vi "UHR-Fleezers Control (host) - Avogadro v3.vi"() -> ()   [LabVIEW 2014] (continued)
            n3132 = call "Calculate MCL scan parameters.vi"("Input parameters"=w5700) -> ("Scan steps(MCL)"=w5699:dbl, "Scan Freq. Increment (MCL)"=w5698:dbl, "MCL Count"=w5697:dbl)
            "MCL Count" <- w5697
            n3133 = xnode "Read/Write Control"("FPGA VI Reference In"=w5714, "error in"=w5713, "Scan steps (MCL)"=w5699, "Number of scans (MCL)"=w5710, "Cycles per step (MCL)"=u64 1, "Scan freq.  increment (MCL)"=w5698, "1D or 2D Scan?"=w5711, "MCL Scan Axis"=w5711, "Cont. Scan (MCL)"=w5711, "MCL count"=w5697) -> ("FPGA VI Reference Out"=w5696:T41, "error out"=w5712:errorcluster)
            n3134 = local write "MCL Scanning"(w5715) -> ()
            n3135 = local write "wait to reset values"(w5715) -> ()
            n3136 = xnode "Read/Write Control"("FPGA VI Reference In"=w5696, "error in"=w5712, "AI to FIFO"=w5715, "APD to FIFO"=w5715, "Start scan"=w5715, "Start scan (MCL)"=w5715) -> ("FPGA VI Reference Out"=w5717:T41, "error out"=w5716:errorcluster)
          }
        }
        "Raster Scanning..." <- TRUE ("Scanning...")
      }
    }
    n3137 = case "Start MCL raster scan" shown="True" w4761 {
      tunnel: w4926 -> [w5558 w5576]
      tunnel: w4925 -> [w5557 w5575]
      tunnel: [w5558 w5571] -> w4877
      tunnel: [w5557 w5570] -> w4876
      tunnel: [FALSE w5569] -> w4909
      tunnel: "Start MCL Scan" -> [_ w5566]
      tunnel: "Confocal Image" -> [_ w5565]
      tunnel: "Confocal Linescan" -> [_ _]
      frame False {
      }
      frame True {
        w5569 = TRUE
        n3138 = case shown="True" "Restart DMA? (MCL)" {
          tunnel: [w5652 w5654] -> w5574
          tunnel: [w5651 w5653] -> w5573
          tunnel: w5576 -> [w5652 w5657]
          tunnel: w5575 -> [w5651 w5656]
          frame False {
          }
          frame True {
            n3139 = call "reset FPGA DMA.vi"("error in"=w5656, "FPGA VI Reference In"=w5657) -> ("error out"=w5653:errorcluster, "FPGA VI Reference Out"=w5654:T41)
            n3140 = local write "Overflow (data lost)"(FALSE ("Overflow (data lost)")) -> ()
          }
        }
        n3141 = case shown="False" w5566 {
          tunnel: w5565 -> [w5579 _]
          frame False {
            n3142 = property on="Confocal Image" class="Bool (strict)"("Value"=FALSE ("Start Confocal Map")) -> ()  [unwired: 2 in, 2 out]
            n3143 = property on="2D or 1D Scan" class="Bool (strict)"("Val(Sgnl)"=w5579) -> ()  [unwired: 2 in, 2 out]
          }
          frame True {
          }
        }
        n3144 = local write "Tab Control 6"(T63."Imaging" ("Tab Control 6")) -> ()
        n3145 = local read "T3 X (V)"() -> (w5561:dbl)
        n3146 = local write "MCL Scanning"(w5569) -> ()
        n3147 = local read "T3 Y (V)"() -> (w5560:dbl)
        n3148 = local read "AO2"() -> (w5562:dbl)
        n3149 = local read "AO1"() -> (w5563:dbl)
        n3150 = case shown="True" "Center Scan" {
          tunnel: w5574 -> [w5592 w5614]
          tunnel: w5573 -> [w5591 w5613]
          tunnel: [w5590 w5612] -> w5571
          tunnel: [w5589 w5611] -> w5570
          tunnel: [w5584 w5608] -> w5568
          tunnel: [w5585 w5607] -> w5567
          tunnel: w5563 -> [w5582 w5610]
          tunnel: w5562 -> [w5581 w5609]
          tunnel: "Scan trap 3 or Fl?" -> [w5587 w5606]
          tunnel: w5561 -> [w5586 w5599]
          tunnel: w5560 -> [w5583 w5600]
          frame False {
            w5588 = TRUE ("AI to FIFO")
            n3151 = case shown="False" w5587 {
              tunnel: [w5594 w5598] -> w5585
              tunnel: w5586 -> [_ w5598]
              tunnel: [w5595 w5597] -> w5584
              tunnel: w5583 -> [_ w5597]
              tunnel: w5582 -> [w5595 _]
              tunnel: w5581 -> [w5594 _]
              tunnel: [FALSE ("AI to FIFO") TRUE ("AI to FIFO")] -> w5580
              frame False {
              }
              frame True {
              }
            }
            n3152 = xnode "Read/Write Control"("FPGA VI Reference In"=w5592, "error in"=w5591, "AI to FIFO"=w5588, "APD to FIFO"=w5588, "Start scan (MCL)"=w5588, "ScanTrap 3 or Fl-laser"=w5580) -> ("FPGA VI Reference Out"=w5590:T41, "error out"=w5589:errorcluster)
          }
          frame True {
            n3153 = local read "Actual MCL Inc (V)"() -> (w5601:dbl)
            n3154 = local read "Scan steps (MCL)"() -> (w5602:u64)
            n3155 = local read "Scan lines (y)"() -> (w5603:u64)
            n3156 = local read "Fast Scan Dir"() -> (w5604:bool)
            n3157 = local read "2D or 1D Scan"() -> (w5605:bool)
            n3158 = case shown="False" w5606 {
              tunnel: w5614 -> [w5632 w5650]
              tunnel: w5613 -> [w5631 w5649]
              tunnel: [w5630 w5648] -> w5612
              tunnel: [w5629 w5647] -> w5611
              tunnel: w5610 -> [w5625 _]
              tunnel: w5609 -> [w5624 _]
              tunnel: [w5622 w5642] -> w5608
              tunnel: [w5621 w5641] -> w5607
              tunnel: w5605 -> [w5620 w5640]
              tunnel: w5604 -> [w5619 w5639]
              tunnel: w5603 -> [w5618 w5638]
              tunnel: w5602 -> [w5617 w5637]
              tunnel: w5601 -> [w5615 w5635]
              tunnel: w5600 -> [_ w5634]
              tunnel: w5599 -> [_ w5633]
              frame False {
                w5628 = TRUE ("AI to FIFO")
                n3159 = Bundle("Actual MCL Inc (V)"=w5615, "Scan steps (MCL)"=w5617, "Scan lines (y)"=w5618, "AO1"=w5625, "AO2"=w5624) -> (w5623:T67)  [unwired: 1 in]
                n3160 = call "Center Scan calculation.vi"("2D or 1D Scan"=w5620, "Fast Scan Dir"=w5619, "Input parameters"=w5623) -> ("X"=w5621:dbl, "Y"=w5622:dbl)
                n3161 = call "Volt to I16.vi"("Voltage In"=w5622) -> ("I16 Voltage Out"=w5627:i16)
                n3162 = call "Volt to I16.vi"("Voltage In"=w5621) -> ("I16 Voltage Out"=w5626:i16)
                n3163 = xnode "Read/Write Control"("FPGA VI Reference In"=w5632, "error in"=w5631, "AI to FIFO"=w5628, "APD to FIFO"=w5628, "Start scan (MCL)"=w5628, "AO1 (Y)"=w5627, "AO2 (X)"=w5626, "ScanTrap 3 or Fl-laser"=FALSE ("AI to FIFO")) -> ("FPGA VI Reference Out"=w5630:T41, "error out"=w5629:errorcluster)
              }
              frame True {
                w5646 = TRUE ("AI to FIFO")
                n3164 = Bundle("Actual MCL Inc (V)"=w5635, "Scan steps (MCL)"=w5637, "Scan lines (y)"=w5638, "T3 Y (V)"=w5634, "T3 X (V)"=w5633) -> (w5643:T68)  [unwired: 1 in]
                n3165 = call "Center Scan calculation.vi"("2D or 1D Scan"=w5640, "Fast Scan Dir"=w5639, "Input parameters"=w5643) -> ("X"=w5641:dbl, "Y"=w5642:dbl)
                n3166 = call "Volt to I16.vi"("Voltage In"=w5642) -> ("I16 Voltage Out"=w5645:i16)
                n3167 = call "Volt to I16.vi"("Voltage In"=w5641) -> ("I16 Voltage Out"=w5644:i16)
                n3168 = xnode "Read/Write Control"("FPGA VI Reference In"=w5650, "error in"=w5649, "AI to FIFO"=w5646, "APD to FIFO"=w5646, "Start scan (MCL)"=w5646, "Piezo Trap Y (AO4)"=w5645, "Piezo Trap X (AO5)"=w5644, "ScanTrap 3 or Fl-laser"=TRUE ("AI to FIFO")) -> ("FPGA VI Reference Out"=w5648:T41, "error out"=w5647:errorcluster)
              }
            }
          }
        }
        "Initial Y" <- w5568
        "Initial X" <- w5567
        "wait to reset values" <- w5569
      }
    }
    n3169 = xnode "Read/Write Control"("FPGA VI Reference In"=w4738) -> ("FPGA VI Reference Out"=w4633:T41, "BD1 Frequency Out 1"=w4740:u64, "Piezo X out"=w4672:i16, "Piezo Y out"=w4671:i16)  [unwired: 1 in, 1 out]
    n3170 = And(x="Save scans", y=w4906) -> (x .and. y?=w4924:bool)
    n3171 = call "IR AOM word to freq.vi"("Frequency Word In (U64)"=w4740) -> ("Frequency Out (MHz)"=w4739:dbl)
    n3172 = Divide(x=w4672, y=w4706) -> (x/y=w4705:dbl)
    n3173 = Divide(x=w4671, y=w4706) -> (x/y=w4704:dbl)
    n3174 = local read "BD 1 Frequency 2 (MHz)"() -> (w4770:dbl)
    n3175 = Subtract(x=w4770, y=w4739) -> (x-y=w4703:dbl)
    "Current deltaF (MHz)" <- w4703
    n3176 = Build Array(w4703, w4705, w4704) -> (w4629:dbl[])
    "Trap position array" <- w4629
    n3177 = control-ref of="Piezo trap cursor control"() -> (w4712:refnum<vi>)
    n3178 = Unbundle By Name("Cursor control") -> ("X"=w4714:bool, "Y"=w4713:bool)
    n3179 = local read "APD Elements/DMA read"() -> (w4801:u32)
    n3180 = local read "Trap AI Elements/DMA read"() -> (w4898:u32)
    n3181 = case shown="False" w4714 {
      tunnel: w4712 -> [w5061 w5071]
      tunnel: w4633 -> [_ w5063]
      frame False {
        n3182 = local read "T3 X (V)"() -> (w5062:dbl)
        n3183 = property class="XYGraph (strict)"(reference=w5061, "Cursor.Cursor X"=w5062) -> ()  [unwired: 1 in, 2 out]
      }
      frame True {
        n3184 = property class="XYGraph (strict)"(reference=w5071) -> ("Cursor.Cursor X"=w5068:dbl)  [unwired: 1 in, 2 out]
        n3185 = In Range and Coerce(upper limit=10.0, x=w5068, lower limit=0.0) -> (coerced(x)=w5066:dbl)  [unwired: 1 out]
        n3186 = Multiply(x=3276.7, y=w5066) -> (x*y=w5065:dbl)
        n3187 = To Unsigned Word Integer(number=w5065) -> (unsigned 16bit integer=w5064:u16)
        n3188 = xnode "Read/Write Control"("FPGA VI Reference In"=w5063, "Piezo Trap X (AO5)"=w5064) -> ()  [unwired: 1 in, 2 out]
      }
    }
    n3189 = case shown="False" w4713 {
      tunnel: w4712 -> [w5048 w5060]
      tunnel: w4633 -> [_ w5051]
      frame False {
        n3190 = local read "T3 Y (V)"() -> (w5050:dbl)
        n3191 = Negate(x=w5050) -> (-x=w5049:dbl)
        n3192 = property class="XYGraph (strict)"(reference=w5048, "Cursor.Cursor Y"=w5049) -> ()  [unwired: 1 in, 2 out]
      }
      frame True {
        n3193 = property class="XYGraph (strict)"(reference=w5060) -> ("Cursor.Cursor Y"=w5057:dbl)  [unwired: 1 in, 2 out]
        n3194 = In Range and Coerce(upper limit=0.0, x=w5057, lower limit=-10.0) -> (coerced(x)=w5056:dbl)  [unwired: 1 out]
        n3195 = Negate(x=w5056) -> (-x=w5054:dbl)
        n3196 = Multiply(x=3276.7, y=w5054) -> (x*y=w5053:dbl)
        n3197 = To Unsigned Word Integer(number=w5053) -> (unsigned 16bit integer=w5052:u16)
        n3198 = xnode "Read/Write Control"("FPGA VI Reference In"=w5051, "Piezo Trap Y (AO4)"=w5052) -> ()  [unwired: 1 in, 2 out]
      }
    }
    n3199 = local read "Trap Pos Elements/DMA read"() -> (w4873:u32)
    n3200 = local read "DMA Update Period (s)"() -> (w4754:dbl)
    n3201 = xnode "Invoke Method"("FPGA VI Reference In"=w4877, "error in"=w4876, "Number of Elements"=w4873, "Timeout (ms)"=-1) -> ("Data"=w4709:u16[], "Elements Remaining"=→"Trap Pos FIFO El Remaining":u32)  [unwired: 2 out]
    n3202 = xnode "Get Trap Data"("FPGA VI Reference In"=w4877, "error in"=w4876, "Number of Elements"=w4898, "Timeout (ms)"=-1 ("Timeout")) -> ("FPGA VI Reference Out"=w4769:T41, "error out"=w4825:errorcluster, "Data"=w4758:i16[], "Elements Remaining"=w4958:u32)
    "FIFO El. Rem." <- w4958
    n3203 = local read "Trap AI FIFO Depth"() -> (w4960:u32)
    n3204 = xnode "Get APD Data"("FPGA VI Reference In"=w4877, "error in"=w4876, "Number of Elements"=w4801, "Timeout (ms)"=-1) -> ("Data"=w4750:u32[], "Elements Remaining"=→"APD FIFO Elements Remaining":u32)  [unwired: 2 out]
    n3205 = feedback #1(0.0) -> (w4871:dbl)
    n3206 = To Time Stamp(1:w4871) -> (0:w4653:timestamp)
    n3207 = Add(x=w4754, y=w4871) -> (x+y=w4935:dbl)
    n3208 = feedback-in #1(w4935) -> ()
    n3209 = Subtract(x=w4960, y=w4898) -> (x-y=w4959:u32)
    n3210 = local read "APD Integration Time (s)"() -> (w4742:dbl)
    n3211 = local read "Scan trap 3 or Fl?"() -> (w4628:bool)
    n3212 = Divide(x=w4958, y=w4959) -> (x/y=w4957:dbl)
    "Buffer Status" <- w4957
    n3213 = local read "Trap Sets"() -> (w4759:u32)
    n3214 = Equal?(x=w4957, y=1.0) -> (x = y?=w4955:bool)
    n3215 = local read "Number of APDs"() -> (w4749:u8)
    n3216 = case "Alert buffer overflow" shown="True" w4955 {
      frame False {
      }
      frame True {
        n3217 = call <vilib>:"Beep.vi"() -> ()  [unwired: 3 in, 9 out]
        "Overflow (data lost)" <- TRUE ("Overflow (data lost)")
      }
    }
    n3218 = call "deinterlace.vi"("Scan trap 3 or Fl?"=w4628, "Detector type"="Detector Type", "Data"=w4758, "Trap sets"=w4759, "Flip x sign"="Flip X Sign") -> ("Channel pattern"=w4755:i32, "Channel names"=w4711:string[], "Deinterlaced normalized data"=w4647:dbl[][], "Deinterlaced data"=w4756:i16[])
    "AI labels" <- w4711
    n3219 = local read "Data Period (s)"() -> (w4646:dbl)
    n3220 = call "Trap_position_vectors.vi"("Data array"=w4709) -> ("Output data for plotting"=w4708:dbl[][], "Output data for saving"=w4707:u64[])
    n3221 = call "APD data extraction.vi"("Data"=w4750, "Number of APD's"=w4749, "APD integration time (s)"=w4742, "APD Ave N"="APD Ave N", "APD Disp. Downsample"="APD Disp. Downsample", "APD Disp. Scale"="APD Disp. Scale", "Time Stamp"=w4653) -> ("Output cluster"=→"APD rates cluster":T2, "Output Data"=w4745:T69, "Output waveform"=w4744:waveform(dbl)[], "APD Display period (s)"=w4743:dbl)
    "APD Display Period (s)" <- w4743
    n3222 = Reciprocal(x=w4743) -> (1/x=→"APD Display Freq. (Hz)":dbl)
    n3223 = Multiply(x=w4646, y="Trap Disp. Downsample") -> (x*y=w4872:dbl)
    "Display Period (s)" <- w4872
    n3224 = for {
      tunnel: w4647 -> [w5086] mode=indexing
      tunnel: [w5085] -> w4710 mode=indexing
      n3225 = call-poly <vilib>:"Mean.vi"("X"=w5086) -> ("mean"=w5085:dbl)  [unwired: 1 out]
    }
    "Values" <- w4710
    n3226 = Decimate 1D Array(w4756) -> (w4863:i16[], w4862:i16[], w4860:i16[], w4859:i16[])  [unwired: 9 out]
    n3227 = call "Generate Waveform.vi"("Downsampling"="Trap Disp. Downsample", "Data Period (s)"=w4646, "Data"=w4647, "Plot names"=w4711, "Time Stamp"=w4653) -> ("Downsampled data"=w4689:waveform(dbl)[], "Non downsampled waveform"=w4751:waveform(dbl)[])
    n3228 = Multiply(x="APD Disp. Scale", y=w4744) -> (x*y=w4881:waveform(dbl)[])
    n3229 = Reciprocal(x=w4872) -> (1/x=→"Trap Disp. Freq. (Hz)":dbl)
    n3230 = Multiply(x="APD Disp. Downsample", y=w4742) -> (x*y=w4880:dbl)
    n3231 = Divide(x=w4863, y=w4862) -> (x/y=w4864:dbl[])
    n3232 = Divide(x=w4860, y=w4859) -> (x/y=w4861:dbl[])
    n3233 = Divide(x=w4881, y=w4880) -> (x/y=w4805:waveform(dbl)[])
    n3234 = case shown="1" "Plot Trap Positions" {
      tunnel: [w5072 w5080] -> w4733
      frame 0, Default {
        n3235 = local read "BD 1 Frequency 2 (MHz)"() -> (w5075:dbl)
        n3236 = local read "BD 1 Frequency 1 (MHz)"() -> (w5076:dbl)
        n3237 = local read "T3 Y (V)"() -> (w5073:dbl)
        n3238 = local read "T3 X (V)"() -> (w5074:dbl)
        n3239 = Build Array(w5076, w5075, w5074, w5073) -> (w5072:dbl[])
      }
      frame 1 {
        w5079 = 60.0
        n3240 = local read "Piezo trap x\noffset (V)"() -> (w5077:dbl)
        n3241 = Build Array(w5079, w5079, w5077, "Piezo trap y\noffset (V)") -> (w5080:dbl[])
      }
    }
    n3242 = Split 1D Array(array=w4864, index="N El. to Ave.") -> (second subarray=w4867:dbl[])  [unwired: 1 out]
    n3243 = Split 1D Array(array=w4861, index="N El. to Ave.") -> (second subarray=w4866:dbl[])  [unwired: 1 out]
    n3244 = case shown="True" "Chart APD?" {
      tunnel: w4805 -> [_ w5026]
      frame False {
      }
      frame True {
        n3245 = Index Array(array=w5026, index=0) -> (element=w5036:waveform(dbl))
        n3246 = Index Array(array=w5026, index=1) -> (element=w5034:waveform(dbl))
        n3247 = Index Array(array=w5026, index=2) -> (element=w5028:waveform(dbl))
        n3248 = Subtract(x=w5036, y="APD 1 Offset") -> (x-y=w5032:waveform(dbl))
        n3249 = Subtract(x=w5034, y="APD 2 Offset") -> (x-y=w5031:waveform(dbl))
        n3250 = Subtract(x=w5028, y="APD 3 Offset") -> (x-y=w5025:waveform(dbl))
        n3251 = Build Array(w5032, w5031, w5025) -> (→"APD Chart":waveform(dbl)[])
      }
    }
    n3252 = local read "AOM X Cal (nm/MHz)"() -> (w4735:dbl)
    n3253 = call-poly <vilib>:"Mean.vi"("X"=w4867) -> ("mean"=w4855:dbl)  [unwired: 1 out]
    n3254 = call-poly <vilib>:"Mean.vi"("X"=w4866) -> ("mean"=w4854:dbl)  [unwired: 1 out]
    n3255 = local read "Trap X AI1 (DMA)"() -> (w4865:T23)
    n3256 = To Fixed-Point(number=w4854) -> (fixed-point=w4852:fxp<+/-,16,1>)  [unwired: 1 in]
    n3257 = To Fixed-Point(number=w4855) -> (fixed-point=w4853:fxp<+/-,16,1>)  [unwired: 1 in]
    n3258 = Bundle By Name(cluster=w4865, "Set 1"=w4853, "Set 2"=w4852) -> (→"Trap X AI1 (DMA)":T23)
    n3259 = Build Array(w4735, w4735, "Piezo Trap X cal (nm/V)", "Piezo Trap Y cal (nm/V)") -> (w4734:dbl[])
    n3260 = Cluster To Array(cluster="Negate Axis") -> (array=w4728:bool[])
    n3261 = call "Generate Trap Positiion Waveform.vi"("Base trap positions"=w4733, "Data Period (s)"=w4646, "Input data"=w4708, "Position calibration values"=w4734, "Trap Pos. Disp. Downsample (s)"="Trap Pos. Disp. Downsample", "Negate axis"=w4728, "Time Stamp"=w4653) -> ("Output waveforms"=w4716:waveform(dbl)[], "Output trap positions"=w4662:cluster{"X":dbl[], "Y":dbl[]}[])  [unwired: 2 in]
    "Trap Positions" <- w4716
    n3262 = Initialize Array(0.0) -> (w4730:dbl[][])  [unwired: 2 in]
    n3263 = local read "Display Period (s)"() -> (w4889:dbl)
    n3264 = for {
      tunnel: w4716 -> [w5084] mode=indexing
      shift-right: [w5082] -> w4718
      shift-left: w4730 -> [w5083]
      n3265 = Unbundle By Name(w5084) -> ("Y"=w5081:dbl[])
      n3266 = Build Array (concatenate)(w5083, w5081) -> (w5082:dbl[][])
    }
    n3267 = Build Array (concatenate)(w4744, w4689) -> (w4753:waveform(dbl)[])
    "All Signals" <- w4753
    n3268 = Initialize Array(0.0) -> (w4643:dbl[][])  [unwired: 2 in]
    n3269 = feedback #2(w4643) -> (w4642:dbl[][])
    n3270 = Divide(x="Bead Sep. Int. Time (s)", y=w4889) -> (x/y=w4724:dbl)
    n3271 = case shown="True" "Start position \nscan" {
      tunnel: w4642 -> [w5039 _]
      tunnel: [w5039 w5047] -> w4641
      tunnel: "T3 positioning test range (V)" -> [_ w5041]
      frame False {
      }
      frame True {
        n3272 = local read "BD 1 Frequency 1 (MHz)"() -> (→"AOM position for scan (MHz)":dbl)
        n3273 = Unbundle By Name(w5041) -> ("Xmin"=w5043:dbl, "Ymin"=w5042:dbl)
        n3274 = local write "Start position \nscan"(FALSE) -> ()
        n3275 = local write "T3 X (V)"(w5043) -> ()
        n3276 = local write "T3 Y (V)"(w5042) -> ()
        n3277 = Initialize Array(0.0) -> (w5047:dbl[][])  [unwired: 2 in]
        "Position\nscanning..." <- TRUE
      }
    }
    n3278 = case shown="True" "Measure \ncorrelation?" {
      tunnel: w4647 -> [_ w5013]
      tunnel: w4646 -> [_ w5012]
      tunnel: w4641 -> [w4983 w4996]
      tunnel: [w4983 w4989] -> w4640
      tunnel: "T3 positioning test range (V)" -> [_ w4988]
      tunnel: w4633 -> [_ w4984]
      frame False {
      }
      frame True {
        n3279 = local read "DMA Update Period (s)"() -> (w4991:dbl)
        n3280 = Divide(x="Correlation integration time (s)", y=w4991) -> (x/y=w4990:dbl)
        n3281 = To Word Integer(number=w4990) -> (16bit integer=w4986:i16)
        n3282 = Divide(x="Correlation integration time (s)", y=w5012) -> (x/y=w5006:dbl)
        n3283 = Initialize Array(0.0, w5006, 4) -> (w5009:dbl[][])
        n3284 = feedback #3(w5009) -> (w5008:dbl[][])
        n3285 = call "correlation calculation for trap 3 absolute positioning.vi"("Number of sets to average"=w5006, "Accumulated array"=w5008, "raw data"=w5013) -> ("Accumulated array out"=w5007:dbl[][], "Y correlation"=w5004:dbl, "X correlation"=w5005:dbl)
        "3-1 x correlation" <- w5005
        "3-1 y correlation" <- w5004
        n3286 = feedback-in #3(w5007) -> ()
        n3287 = Increment(x=w4986) -> (x+1=w4985:i16)
        n3288 = local read "Position\nscanning..."() -> (w4995:bool)
        n3289 = Bundle("X correlation"=w5005, "Y correlation"=w5004) -> (w5003:T70)  [unwired: 1 in]
        n3290 = local read "T3 Y (V)"() -> (w5001:dbl)
        n3291 = local read "T3 X (V)"() -> (w5002:dbl)
        n3292 = Bundle("T3 X (V)"=w5002, "T3 Y (V)"=w5001) -> (w5000:cluster{"T3 X (V)":dbl, "T3 Y (V)":dbl})  [unwired: 1 in]
        n3293 = feedback #4(i16 0) -> (w4998:i16)
        n3294 = call "correlation scan.vi"("Correlations in"=w5003, "Voltages in"=w5000, "Cycle counter"=w4998, "in put Array"=w4996, "T3 positioning \ntest range (V)"=w4988, "Number of acquisition cycles"=w4985, "Scanning?"=w4995) -> ("Voltages out"=w4993:cluster{"X":dbl, "Y":dbl}, "Scanning out"=w4994:bool, "Output array"=w4989:dbl[][], "Cycle counter out"=w4997:i16)
        n3295 = feedback-in #4(w4997) -> ()
        n3296 = local write "Position\nscanning..."(w4994) -> ()
        n3297 = case shown="True" w4994 {
          tunnel: w4993 -> [_ w5024]
          tunnel: w4984 -> [_ w5018]
          frame False {
          }
          frame True {
            w5022 = 3276.7
            n3298 = Unbundle By Name(w5024) -> ("X"=w5023:dbl, "Y"=w5021:dbl)
            n3299 = Multiply(x=w5022, y=w5023) -> (x*y=w5020:dbl)
            n3300 = Multiply(x=w5022, y=w5021) -> (x*y=w5019:dbl)
            n3301 = To Word Integer(number=w5020) -> (16bit integer=w5017:i16)
            n3302 = To Word Integer(number=w5019) -> (16bit integer=w5016:i16)
            n3303 = local write "T3 Y (V)"(w5021) -> ()
            n3304 = local write "T3 X (V)"(w5023) -> ()
            n3305 = xnode "Read/Write Control"("FPGA VI Reference In"=w5018, "Piezo Trap X (AO5)"=w5017, "Piezo Trap Y (AO4)"=w5016) -> ()  [unwired: 1 in, 2 out]
          }
        }
        n3306 = case shown="True" "Stop scan" {
          frame False {
          }
          frame True {
            n3307 = local write "Position\nscanning..."(FALSE) -> ()
            n3308 = local write "Stop scan"(FALSE) -> ()
          }
        }
      }
    }
    n3309 = feedback-in #2(w4640) -> ()
    n3310 = feedback #5(w4718) -> (w4725:dbl[][])
    n3311 = call "Trap Pos RMS.vi"("Accumulated array"=w4725, "New Array"=w4718, "Number of sets to average"=w4724) -> ("Output accumulated array"=w4723:dbl[][], "RMS"=w4721:dbl[], "Mean"=w4722:dbl[])
    n3312 = feedback-in #5(w4723) -> ()
    n3313 = Index Array(array=w4718, index (row)=0 ("index")) -> (element=w4717:dbl[])  [unwired: 1 in]
    n3314 = local read "Two Trap Offset Values"() -> (w4699:T32)
    n3315 = Array To Cluster(array=w4721) -> (cluster=→"Trap RMS (ang)":T71)
    n3316 = Array To Cluster(array=w4722) -> (cluster=→"Mean Trap Positions (nm)":T72)
    n3317 = local read "MCL offset scanning range (V)"() -> (w4697:T4)
    n3318 = local read "Multi-MCL offset array"() -> (w4698:T31)
    n3319 = local read "Multiple-MCL offset?"() -> (w4702:bool)
    n3320 = local read "Offset file step size"() -> (w4700:dbl)
    n3321 = local read "T1 calibration"() -> (w4696:T12)
    n3322 = local read "T2 calibration"() -> (w4695:T12)
    n3323 = local read "T3 calibration"() -> (w4694:T12)
    n3324 = local read "Trap Disp. Downsample"() -> (w4651:dbl)
    n3325 = Build Array(w4696, w4695, w4694) -> (w4693:T56)
    n3326 = call "calibrate trap data V3RG.vi"("array of calibration clusters"=w4693, "Trap position array"=w4629, "MCL offset scanning range (V)"=w4697, "Multi-MCL offset array"=w4698, "two trap offset values"=w4699, "Dynamic offset update"="Dynamic offset\nupdate", "Multiple-MCL offset?"=w4702, "x (true) or y (false)"=TRUE, "Data array"=w4689, "Offset File step size"=w4700) -> ("Positions out"=w4691:dbl[][], "Forces out (pN)"=w4690:dbl[][])
    n3327 = local read "Mean Trap Positions (nm)"() -> (w4688:T6)
    n3328 = local read "Trap 2 Bead Size (nm)"() -> (w4666:dbl)
    n3329 = local read "Trap 3 Bead Size (nm)"() -> (w4665:dbl)
    n3330 = local read "Trap 1 Bead Size (nm)"() -> (w4667:dbl)
    n3331 = case shown="True" "Measure \ncorrelation?" {
      tunnel: w4640 -> [_ w4967]
      tunnel: "T3 positioning test range (V)" -> [_ w4966]
      frame False {
      }
      frame True {
        n3332 = Unbundle By Name(w4966) -> ("Xmax"=w4970:dbl, "Xmin"=w4971:dbl, "increment"=w4976:dbl, "Ymax"=w4972:dbl, "Ymin"=w4973:dbl)
        n3333 = Index Array(array=w4967, index (col)=3) -> (element=w4969:dbl[])  [unwired: 1 in]
        n3334 = Index Array(array=w4967, index (col)=2) -> (element=w4968:dbl[])  [unwired: 1 in]
        n3335 = Subtract(x=w4972, y=w4973) -> (x-y=w4975:dbl)
        n3336 = Subtract(x=w4970, y=w4971) -> (x-y=w4974:dbl)
        n3337 = Quotient & Remainder(x=w4975, y=w4976) -> (floor(x/y)=w4978:dbl)  [unwired: 1 out]
        n3338 = Quotient & Remainder(x=w4974, y=w4976) -> (floor(x/y)=w4977:dbl)  [unwired: 1 out]
        n3339 = Increment(x=w4977) -> (x+1=w4980:dbl)
        n3340 = Increment(x=w4978) -> (x+1=w4979:dbl)
        n3341 = Reshape Array(w4969, w4980, w4979) -> (→"Correlations in Y":dbl[][])
        n3342 = Reshape Array(w4968, w4980, w4979) -> (→"Correlations in X":dbl[][])
      }
    }
    n3343 = local read "Data Period (s)"() -> (w4655:dbl)
    n3344 = Index Array(array=w4689, index="index 2") -> (element=w4800:waveform(dbl))
    n3345 = Index Array(array=w4689, index="index 1") -> (element=w4796:waveform(dbl))
    n3346 = Multiply(x=w4651, y=w4655) -> (x*y=w4654:dbl)
    n3347 = Unbundle By Name(w4800) -> ("Y"=w4799:dbl[])
    n3348 = Unbundle By Name(w4796) -> ("Y"=w4795:dbl[])
    n3349 = Build Array(w4667, w4666, w4665) -> (w4664:dbl[])
    n3350 = call "Force and position waveforms.vi"("Input waveforms"=w4689, "Forces  (pN)"=w4690, "Deflections (nm)"=w4691, "Mean Trap Positions (nm)"=w4688) -> ("1D data"=w4674:waveform(dbl)[], "Absolute Positions"=w4670:waveform(dbl)[], "Forces"=w4648:waveform(dbl)[], "Deflections"=w4669:waveform(dbl)[], "Raw Data"=w4668:waveform(dbl)[])
    n3351 = call-poly <vilib>:"Mean.vi"("X"=w4795) -> ("mean"=→"Trap 1 sum mean":dbl)  [unwired: 1 out]
    n3352 = call-poly <vilib>:"Mean.vi"("X"=w4799) -> ("mean"=→"Trap 2 sum mean":dbl)  [unwired: 1 out]
    n3353 = local read "Trap 3 Bead Size (nm)"() -> (w4638:dbl)
    n3354 = call "2D force plotting.vi"("Trap positions"=w4662, "Calibration"="2D force calibration", "Bead sizes"=w4664, "Raw Data"=w4668, "Deflections"=w4669, "Forces"=w4648, "Absolute Positions"=w4670) -> ("Output waveforms"=→"2D forces":waveform(dbl)[], "Output"=→"2D values (force/position/raw)":T1, "Junctions"=w4660:cluster{"X":dbl[], "Y":dbl[]}[], "deflection lines"=w4661:cluster{"X":dbl[], "Y":dbl[]}[], "tether sizes"=w4656:dbl[][])
    n3355 = local read "Trap 2 Bead Size (nm)"() -> (w4676:dbl)
    n3356 = local read "Trap 1 Bead Size (nm)"() -> (w4677:dbl)
    n3357 = call "2D tether waveforms.vi"("tether sizes"=w4656, "Data period (s)"=w4654, "Time Stamp"=w4653, "Forces"=w4648) -> ("tethers"=→"2D tethers":waveform(dbl)[], "output forces"=→"tether forces":waveform(dbl)[], "Output Means"=→"Output Means":T9)  [unwired: 2 in]
    n3358 = call "1D force plotting.vi"("Calibration"="Calibration", "Forces"=w4648, "Deflections"=w4669, "Raw Data"=w4668, "Only check fixed trap T2"="Only check fixed trap T2") -> ("Vec Mean of T1 T2"=→"Vec Mean of T1 T2":dbl[], "Output force values"=w4683:T73, "Output waveforms"=→"Force":waveform(dbl)[])
    n3359 = call "1D bead separation calculation.vi"("Trap 1 Bead Size (nm)"=w4677, "Trap 2 Bead Size (nm)"=w4676, "Trap 3 Bead Size (nm)"=w4638, "Absolute Positions"=w4670, "Pair choice"="Pair to \nanalyze") -> ("Output separation"=w4675:dbl[], "Output waveforms"=w4635:waveform(dbl)[])
    "Bead Separation" <- w4635
    n3360 = Build Array (concatenate)(w4662, w4661, w4660) -> (→"Positions \nand displacements":cluster{"X":dbl[], "Y":dbl[]}[])
    n3361 = Unbundle By Name(w4683) -> ("T1 X"=→"T1 X":dbl, "T2 X"=→"T2 X":dbl, "Mean"=w4680:dbl, "Difference"=→"Difference":dbl)
    "Mean" <- w4680
    n3362 = Subtract(x=w4675, y="Offset (nm)") -> (x-y=w4892:dbl[])
    n3363 = feedback #6(w4892) -> (w4891:dbl[])
    n3364 = Build Array (concatenate)(w4892, w4891) -> (w4784:dbl[])
    n3365 = Split 1D Array(array=w4784, index=w4724) -> (first subarray=w4785:dbl[])  [unwired: 1 out]
    n3366 = feedback-in #6(w4785) -> ()
    n3367 = Index Array(array=w4635, index=0) -> (element=w4634:waveform(dbl))
    n3368 = call-poly <vilib>:"Mean.vi"("X"=w4785) -> ("mean"=w4888:dbl)  [unwired: 1 out]
    "Bead Mean (nm)" <- w4888
    n3369 = Build Array (concatenate)(w4674, w4634) -> (w4687:waveform(dbl)[])
    n3370 = Subtract(x=w4785, y=w4888) -> (x-y=w4887:dbl[])
    n3371 = Square(x=w4887) -> (x^2=w4886:dbl[])
    n3372 = call-poly <vilib>:"Mean.vi"("X"=w4886) -> ("mean"=w4885:dbl)  [unwired: 1 out]
    n3373 = Square Root(x=w4885) -> (sqrt(x)=w4884:dbl)
    n3374 = Multiply(x=10.0, y=w4884) -> (x*y=→"RMS (Ang)":dbl)
    n3375 = local read "Data points/scans (MCL)"() -> (w4918:dbl)
    n3376 = Unbundle(w4745) -> ("APD 1"=w4804:u32[])  [unwired: 2 out]
    n3377 = To Double Precision Float(number=w4804) -> (double precision float=w4893:dbl[])
    n3378 = Increment(x=w4918) -> (x+1=w4919:dbl)
    n3379 = feedback #7(w4919) -> (w4922:dbl)
    n3380 = Select(t=0, s=w4909, f=w4922) -> (s? t:f=w4915:dbl)
    n3381 = Array Size(array=w4893) -> (size(s)=w4921:i32)
    n3382 = Add(x=w4921, y=w4915) -> (x+y=w4916:dbl)
    n3383 = Greater?(x=w4916, y=w4918) -> (0:w4917:bool)
    n3384 = local read "MCL Scanning"() -> (w4912:bool)
    n3385 = Select(t=w4915, s=w4917, f=w4916) -> (s? t:f=w4914:dbl)
    n3386 = feedback-in #7(w4914) -> ()
    n3387 = Not(x=w4917) -> (.not. x?=w4911:bool)
    n3388 = And(x=w4911, y=w4912) -> (x .and. y?=w4913:bool)
    n3389 = Or(x=w4913, y=w4909) -> (x .or. y?=w4910:bool)
    n3390 = Equal?(x="Tab Control 6", y=T62."High Res Display") -> (x = y?=w4895:bool)
    n3391 = case "For displaying the high resolution display (no downsampling)" shown="True" w4895 {
      tunnel: w4751 -> [_ w5339]
      frame False {
      }
      frame True {
        n3392 = Index Array(array=w5339, index="High Res. Display") -> (element=w5340:waveform(dbl))
        n3393 = call <vilib>:"Std Deviation and Variance.vi"("X"=w5340) -> ("mean"=w5347:dbl, "standard deviation"=w5352:dbl)  [unwired: 1 in, 1 out]
        "Mean Intensity" <- w5347
        "Sigma" <- w5352
        n3394 = Subtract(x=w5340, y=w5347) -> (x-y=w5346:waveform(dbl))
        n3395 = Select(t=w5346, s="Subtract mean", f=w5340) -> (s? t:f=→"1 Channel":waveform(dbl))
        n3396 = Divide(x=w5352, y=w5347) -> (x/y=→"Sigma/Mean":dbl)
        n3397 = feedback #8(1) -> (w5341:i32)
        n3398 = Greater Or Equal?(x=w5341, y="Slow mean N ave.") -> (x >= y?=w5354:bool)
        n3399 = Increment(x=w5341) -> (x+1=w5356:i32)
        n3400 = Select(t=1, s=w5354, f=w5356) -> (s? t:f=w5343:i32)
        n3401 = feedback-in #8(w5343) -> ()
        n3402 = feedback #9() -> (w5344:waveform(dbl))  [unwired: 1 out]
        n3403 = case shown="Default" w5341 {
          tunnel: [w5359 w5362] -> w5345
          tunnel: w5344 -> [w5361 _]
          tunnel: w5340 -> [w5360 w5362]
          frame Default {
            n3404 = call-poly <vilib>:"Append Waveforms.vi"("waveform B"=w5360, "waveform A"=w5361) -> ("waveform out"=w5359:waveform(dbl))  [unwired: 1 in, 8 out]
          }
          frame 1 {
          }
        }
        n3405 = feedback-in #9(w5345) -> ()
        n3406 = case shown="True" w5354 {
          tunnel: w5345 -> [_ w5358]
          frame False {
          }
          frame True {
            n3407 = call-poly <vilib>:"Mean.vi"("X"=w5358) -> ("mean"=→"Slow mean":dbl)  [unwired: 1 out]
          }
        }
      }
    }
    n3408 = case "For plotting results of scanning MCL (fluorescence and detection laser images)" shown="True" w4910 {
      tunnel: w4909 -> [_ w5418]
      tunnel: w4918 -> [_ _]
      tunnel: w4751 -> [_ w5514]
      tunnel: w4878 -> [_ w5446]
      tunnel: w4745 -> [_ w5424]
      frame False {
      }
      frame True {
        # "Modified by Ronen \nbecause we do not have\nthe license for the\ntwo last image \nmanipulation VI's"
        n3409 = local read "Scan trap 3 or Fl?"() -> (w5402:bool)
        n3410 = case shown="True" w5402 {
          tunnel: [10 ("index") 0 ("index")] -> w5521
          tunnel: [11 ("index") 1 ("index")] -> w5518
          frame False {
          }
          frame True {
          }
        }
        n3411 = Unbundle(w5424) -> ("APD 1"=w5423:u32[], "APD 2"=w5421:u32[], "APD 3"=w5419:u32[])
        n3412 = To Double Precision Float(number=w5423) -> (double precision float=w5422:dbl[])
        n3413 = To Double Precision Float(number=w5421) -> (double precision float=w5420:dbl[])
        n3414 = To Double Precision Float(number=w5419) -> (double precision float=w5412:dbl[])
        n3415 = Index Array(array=w5514, index=w5521) -> (element=w5520:waveform(dbl))
        n3416 = Index Array(array=w5514, index=w5518) -> (element=w5517:waveform(dbl))
        n3417 = local read "Cycles/step (MCL)"() -> (w5476:u64)
        n3418 = Index Array(array=w5514, index="Channel") -> (element=w5516:waveform(dbl))
        n3419 = Unbundle(w5446) -> ("New Image"=w5445:T8, "New Image"=w5444:T8, "New Image"=w5425:T8, "New Image"=w5426:T8, "New Image"=w5427:T8)
        n3420 = local read "Scan steps (MCL)"() -> (w5414:u64)
        n3421 = Unbundle By Name(w5520) -> ("Y"=w5478:dbl[])
        n3422 = Unbundle By Name(w5517) -> ("Y"=w5480:dbl[])
        n3423 = local read "Scan lines (y)"() -> (w5415:u64)
        n3424 = local read "N APD Samp/step"() -> (w5417:dbl)
        n3425 = Unbundle By Name(w5516) -> ("Y"=w5485:dbl[])
        n3426 = call "downsample 1D array - double.vi"("Ave N"=w5476, "Array In"=w5478) -> ("Array Out"=w5477:dbl[])  [unwired: 1 out]
        n3427 = call "downsample 1D array - double.vi"("Ave N"=w5476, "Array In"=w5480) -> ("Array Out"=w5479:dbl[])  [unwired: 1 out]
        n3428 = call "downsample 1D array - double.vi"("Ave N"=w5476, "Array In"=w5485) -> ("Array Out"=w5484:dbl[])  [unwired: 1 out]
        n3429 = Multiply(x=w5414, y=u64 2) -> (x*y=w5416:u64)
        n3430 = feedback #10(w5420) -> (w5464:dbl[])
        n3431 = Build Array (concatenate)(w5464, w5420) -> (w5463:dbl[])
        n3432 = feedback #11(w5412) -> (w5413:dbl[])
        n3433 = Build Array (concatenate)(w5413, w5412) -> (w5411:dbl[])
        n3434 = Select(t=w5420, s=w5418, f=w5463) -> (s? t:f=w5448:dbl[])
        n3435 = feedback-in #10(w5448) -> ()
        n3436 = Select(t=w5412, s=w5418, f=w5411) -> (s? t:f=w5429:dbl[])
        n3437 = feedback-in #11(w5429) -> ()
        n3438 = feedback #12(w5422) -> (w5539:dbl[])
        n3439 = Build Array (concatenate)(w5539, w5422) -> (w5522:dbl[])
        n3440 = Select(t=w5422, s=w5418, f=w5522) -> (s? t:f=w5526:dbl[])
        n3441 = feedback-in #12(w5526) -> ()
        n3442 = feedback #13(w5477) -> (w5528:dbl[])
        n3443 = Build Array (concatenate)(w5528, w5477) -> (w5519:dbl[])
        n3444 = feedback #14(w5484) -> (w5537:dbl[])
        n3445 = Build Array (concatenate)(w5537, w5484) -> (w5536:dbl[])
        n3446 = feedback #15(w5479) -> (w5530:dbl[])
        n3447 = Build Array (concatenate)(w5530, w5479) -> (w5531:dbl[])
        n3448 = Select(t=w5477, s=w5418, f=w5519) -> (s? t:f=w5481:dbl[])
        n3449 = feedback-in #13(w5481) -> ()
        n3450 = Select(t=w5484, s=w5418, f=w5536) -> (s? t:f=w5483:dbl[])
        n3451 = feedback-in #14(w5483) -> ()
        n3452 = Select(t=w5479, s=w5418, f=w5531) -> (s? t:f=w5482:dbl[])
        n3453 = feedback-in #15(w5482) -> ()
        n3454 = call "integrate 1D array interval - double.vi"("Ave N"=w5417, "Array In"=w5448) -> ("Array Out"=w5459:dbl[])  [unwired: 1 out]
        n3455 = call "integrate 1D array interval - double.vi"("Ave N"=w5417, "Array In"=w5429) -> ("Array Out"=w5440:dbl[])  [unwired: 1 out]
        n3456 = call "integrate 1D array interval - double.vi"("Ave N"=w5417, "Array In"=w5526) -> ("Array Out"=w5525:dbl[])  [unwired: 1 out]
        n3457 = Array Size(array=w5459) -> (size(s)=w5460:i32)
        n3458 = Array Size(array=w5440) -> (size(s)=w5441:i32)
        n3459 = Array Size(array=w5525) -> (size(s)=w5527:i32)
        n3460 = Multiply(x=w5415, y=w5416) -> (x*y=w5462:u64)
        n3461 = Multiply(x=w5415, y=w5416) -> (x*y=w5443:u64)
        n3462 = Multiply(x=w5415, y=w5416) -> (x*y=w5535:u64)
        n3463 = Subtract(x=w5462, y=w5460) -> (x-y=w5453:u64)
        n3464 = call-poly <vilib>:"Mean.vi"("X"=w5459) -> ("mean"=w5450:dbl)  [unwired: 1 out]
        n3465 = Subtract(x=w5443, y=w5441) -> (x-y=w5434:u64)
        n3466 = call-poly <vilib>:"Mean.vi"("X"=w5440) -> ("mean"=w5431:dbl)  [unwired: 1 out]
        n3467 = Subtract(x=w5535, y=w5527) -> (x-y=w5475:u64)
        n3468 = call-poly <vilib>:"Mean.vi"("X"=w5525) -> ("mean"=w5472:dbl)  [unwired: 1 out]
        n3469 = call-poly <vilib>:"Mean.vi"("X"=w5481) -> ("mean"=w5465:dbl)  [unwired: 1 out]
        n3470 = call-poly <vilib>:"Mean.vi"("X"=w5483) -> ("mean"=w5470:dbl)  [unwired: 1 out]
        n3471 = call-poly <vilib>:"Mean.vi"("X"=w5482) -> ("mean"=w5468:dbl)  [unwired: 1 out]
        n3472 = Initialize Array(1.0 ("element"), w5453) -> (w5449:dbl[])
        n3473 = Initialize Array(1.0 ("element"), w5434) -> (w5430:dbl[])
        n3474 = Initialize Array(1.0 ("element"), w5475) -> (w5466:dbl[])
        n3475 = Multiply(x=w5449, y=w5450) -> (x*y=w5451:dbl[])
        n3476 = Multiply(x=w5430, y=w5431) -> (x*y=w5432:dbl[])
        n3477 = Multiply(x=w5466, y=w5472) -> (x*y=w5473:dbl[])
        n3478 = Multiply(x=w5466, y=w5468) -> (x*y=w5469:dbl[])
        n3479 = Multiply(x=w5466, y=w5470) -> (x*y=w5471:dbl[])
        n3480 = Multiply(x=w5466, y=w5465) -> (x*y=w5467:dbl[])
        n3481 = Build Array (concatenate)(w5459, w5451) -> (w5461:dbl[])
        n3482 = Build Array (concatenate)(w5440, w5432) -> (w5442:dbl[])
        n3483 = Build Array (concatenate)(w5525, w5473) -> (w5534:dbl[])
        n3484 = Build Array (concatenate)(w5481, w5467) -> (w5529:dbl[])
        n3485 = Build Array (concatenate)(w5483, w5471) -> (w5533:dbl[])
        n3486 = Build Array (concatenate)(w5482, w5469) -> (w5532:dbl[])
        n3487 = Reshape Array(w5461, w5415, w5416) -> (w5457:dbl[][])
        n3488 = Reshape Array(w5442, w5415, w5416) -> (w5438:dbl[][])
        n3489 = Reshape Array(w5534, w5415, w5416) -> (w5512:dbl[][])
        n3490 = Reshape Array(w5529, w5415, w5416) -> (w5495:dbl[][])
        n3491 = Reshape Array(w5533, w5415, w5416) -> (w5487:dbl[][])
        n3492 = Reshape Array(w5532, w5415, w5416) -> (w5502:dbl[][])
        n3493 = Array Subset(array=w5457, index (col)=0 ("index"), length (col)=w5414) -> (w5456:dbl[][])  [unwired: 2 in]
        n3494 = Array Subset(array=w5457, index (col)=w5414) -> (w5454:dbl[][])  [unwired: 3 in]
        n3495 = Array Subset(array=w5438, index (col)=0 ("index"), length (col)=w5414) -> (w5437:dbl[][])  [unwired: 2 in]
        n3496 = Array Subset(array=w5438, index (col)=w5414) -> (w5435:dbl[][])  [unwired: 3 in]
        n3497 = Array Subset(array=w5502, index (col)=0 ("index"), length (col)=w5414) -> (w5507:dbl[][])  [unwired: 2 in]
        n3498 = Array Subset(array=w5502, index (col)=w5414) -> (w5505:dbl[][])  [unwired: 3 in]
        n3499 = Array Subset(array=w5512, index (col)=0 ("index"), length (col)=w5414) -> (w5511:dbl[][])  [unwired: 2 in]
        n3500 = Array Subset(array=w5512, index (col)=w5414) -> (w5509:dbl[][])  [unwired: 3 in]
        n3501 = Array Subset(array=w5487, index (col)=0 ("index"), length (col)=w5414) -> (w5493:dbl[][])  [unwired: 2 in]
        n3502 = Array Subset(array=w5487, index (col)=w5414) -> (w5491:dbl[][])  [unwired: 3 in]
        n3503 = Array Subset(array=w5495, index (col)=0 ("index"), length (col)=w5414) -> (w5500:dbl[][])  [unwired: 2 in]
        n3504 = Array Subset(array=w5495, index (col)=w5414) -> (w5498:dbl[][])  [unwired: 3 in]
        n3505 = for {
          tunnel: w5456 -> [w5547] mode=indexing
          tunnel: [w5546] -> w5455 mode=indexing
          workers-P: _ -> [_]
          n3506 = Reverse 1D Array(array=w5547) -> (reversed array=w5546:dbl[])
        }
        n3507 = for {
          tunnel: w5437 -> [w5545] mode=indexing
          tunnel: [w5544] -> w5436 mode=indexing
          workers-P: _ -> [_]
          n3508 = Reverse 1D Array(array=w5545) -> (reversed array=w5544:dbl[])
        }
        n3509 = for {
          tunnel: w5507 -> [w5553] mode=indexing
          tunnel: [w5552] -> w5506 mode=indexing
          workers-P: _ -> [_]
          n3510 = Reverse 1D Array(array=w5553) -> (reversed array=w5552:dbl[])
        }
        n3511 = for {
          tunnel: w5511 -> [w5555] mode=indexing
          tunnel: [w5554] -> w5510 mode=indexing
          workers-P: _ -> [_]
          n3512 = Reverse 1D Array(array=w5555) -> (reversed array=w5554:dbl[])
        }
        n3513 = for {
          tunnel: w5493 -> [w5549] mode=indexing
          tunnel: [w5548] -> w5492 mode=indexing
          workers-P: _ -> [_]
          n3514 = Reverse 1D Array(array=w5549) -> (reversed array=w5548:dbl[])
        }
        n3515 = for {
          tunnel: w5500 -> [w5551] mode=indexing
          tunnel: [w5550] -> w5499 mode=indexing
          workers-P: _ -> [_]
          n3516 = Reverse 1D Array(array=w5551) -> (reversed array=w5550:dbl[])
        }
        n3517 = Index Array(array=w5512, index (row)=0) -> (element=→"Waveform Graph":dbl[])  [unwired: 1 in]
        n3518 = Add(x=w5455, y=w5454) -> (x+y=w5447:dbl[][])
        n3519 = Add(x=w5436, y=w5435) -> (x+y=w5428:dbl[][])
        n3520 = Add(x=w5506, y=w5505) -> (x+y=w5504:dbl[][])
        n3521 = Add(x=w5510, y=w5509) -> (x+y=w5486:dbl[][])
        n3522 = Add(x=w5492, y=w5491) -> (x+y=w5490:dbl[][])
        n3523 = Add(x=w5499, y=w5498) -> (x+y=w5497:dbl[][])
        n3524 = Divide(x=w5490, y=2) -> (x/y=w5488:dbl[][])
        n3525 = Divide(x=w5504, y=2) -> (x/y=w5405:dbl[][])
        n3526 = To Single Precision Float(number=w5486) -> (single precision float=w5409:sgl[][])
        n3527 = To Single Precision Float(number=w5447) -> (single precision float=w5404:sgl[][])
        n3528 = To Single Precision Float(number=w5428) -> (single precision float=w5403:sgl[][])
        n3529 = Divide(x=w5497, y=2) -> (x/y=w5406:dbl[][])
        n3530 = Transpose 2D Array(2D array=w5488) -> (transposed array=→"Data map":dbl[][])
        n3531 = To Single Precision Float(number=w5405) -> (single precision float=w5408:sgl[][])
        n3532 = To Single Precision Float(number=w5406) -> (single precision float=w5407:sgl[][])
        n3533 = call "IMAQ ArrayToImage"("Image Pixels (Float)"=w5409, "Image"=w5445) -> ("Image Out"=→"APD 1":T8)  [unwired: 8 in, 1 out]
        n3534 = call "IMAQ ArrayToImage"("Image Pixels (Float)"=w5404, "Image"=w5444) -> ("Image Out"=→"APD 2":T8)  [unwired: 8 in, 1 out]
        n3535 = call "IMAQ ArrayToImage"("Image Pixels (Float)"=w5403, "Image"=w5425) -> ("Image Out"=→"APD 3":T8)  [unwired: 8 in, 1 out]
        n3536 = call "IMAQ ArrayToImage"("Image Pixels (Float)"=w5407, "Image"=w5427) -> ("Image Out"=→"Detection Laser Y":T8)  [unwired: 8 in, 1 out]
        n3537 = call "IMAQ ArrayToImage"("Image Pixels (Float)"=w5408, "Image"=w5426) -> ("Image Out"=→"Detection Laser X":T8)  [unwired: 8 in, 1 out]
      }
    }
    n3538 = case "For computing FFTs for display" shown="True" "Compute FFT" {
      tunnel: w4751 -> [_ w5752]
      frame False {
      }
      frame True {
        n3539 = Build Array("FFT 1 Choice 1", "FFT 1 Choice 2", "FFT 2 Choice 1", "FFT 2 Choice 2") -> (w5745:u16[])
        n3540 = Array Size(array=w5752) -> (size(s)=w5751:i32)
        n3541 = feedback-in #16(w5745) -> ()
        n3542 = feedback #16(u16[] [100, 100, 100, 100]) -> (w5746:u16[])
        n3543 = feedback-in #17("# Spectra to Ave.") -> ()
        n3544 = feedback #17("# Spectra to Ave.") -> (w5743:dbl)
        n3545 = Not Equal?(x="# Spectra to Ave.", y=w5743) -> (x != y?=w5742:bool)
        n3546 = Not Equal?(x=w5745, y=w5746) -> (x != y?=w5744:bool)
        n3547 = feedback #18(1.0) -> (w5729:dbl)
        n3548 = Compound Arithmetic op=OR("Reset FFT", w5744, w5742) -> (w5727:bool)
        n3549 = Select(t=1.0, s=w5727, f=w5729) -> (s? t:f=w5731:dbl)
        n3550 = Greater?(x=w5731, y="# Spectra to Ave.") -> (0:w5750:bool)
        n3551 = Increment(x=w5731) -> (x+1=w5730:dbl)
        n3552 = feedback-in #18(w5730) -> ()
        n3553 = local read "DMA Update Period (s)"() -> (w5725:dbl)
        n3554 = Multiply(x="# Spectra to Ave.", y=w5725) -> (x*y=→"Ave. Time (s)":dbl)
        n3555 = Build Array(cluster{"f0":dbl, "df":dbl, "magnitude":dbl[]} {"f0"=0.0, "df"=0.0, "magnitude"=[]} ("PSD")) -> (w5734:cluster{"f0":dbl, "df":dbl, "magnitude":dbl[]}[])
        n3556 = Build Array(w5734, w5734, w5734, w5734) -> (w5736:T74)
        n3557 = feedback #19(w5736) -> (w5741:T74)
        n3558 = for {
          N: 4 -> [_]
          tunnel: w5745 -> [w5774] mode=indexing
          tunnel: w5752 -> [w5775]
          tunnel: w5751 -> [w5777]
          tunnel: w5727 -> [w5770]
          tunnel: w5750 -> [w5769]
          tunnel: "# Spectra to Ave." -> [w5768]
          tunnel: [w5767] -> w5740 mode=indexing
          tunnel: w5741 -> [w5772] mode=indexing
          tunnel: [w5771] -> w5728 mode=indexing
          tunnel: w5731 -> [w5766]
          n3559 = Less?(x=w5774, y=w5777) -> (x < y?=w5776:bool)
          n3560 = Index Array(array=w5775, index=w5774) -> (element=w5773:waveform(dbl))
          n3561 = case shown="True" w5776 {
            tunnel: w5773 -> [_ w5794]
            tunnel: w5772 -> [w5779 w5792]
            tunnel: [w5779 w5780] -> w5771
            tunnel: w5770 -> [_ w5791]
            tunnel: w5769 -> [_ w5784]
            tunnel: w5768 -> [_ w5783]
            tunnel: [cluster{"f0":dbl, "df":dbl, "magnitude":dbl[]} {"f0"=0.0, "df"=0.0, "magnitude"=[]} ("PSD") w5785] -> w5767
            tunnel: w5766 -> [_ w5782]
            frame False {
            }
            frame True {
              n3562 = call <vilib>:"Std Deviation and Variance.vi"("X"=w5794) -> ("mean"=w5795:dbl)  [unwired: 1 in, 2 out]
              n3563 = Subtract(x=w5794, y=w5795) -> (x-y=w5793:waveform(dbl))
              n3564 = xnode "Spectral Measurements"("Signals"=w5793) -> ("PSD"=w5787:cluster{"f0":dbl, "df":dbl, "magnitude":dbl[]})  [unwired: 1 in, 1 out]
              n3565 = case shown="False" w5791 {
                tunnel: w5792 -> [w5804 _]
                tunnel: [w5800 w5809] -> w5780
                tunnel: w5787 -> [w5803 w5810]
                tunnel: w5784 -> [w5802 _]
                frame False {
                  n3566 = Build Array (concatenate)(w5804, w5803) -> (w5801:cluster{"f0":dbl, "df":dbl, "magnitude":dbl[]}[])
                  n3567 = case shown="True" w5802 {
                    tunnel: w5801 -> [w5805 w5808]
                    tunnel: [w5805 w5806] -> w5800
                    frame False {
                    }
                    frame True {
                      n3568 = Delete From Array(array=w5808, index=0) -> (array with subset deleted=w5806:cluster{"f0":dbl, "df":dbl, "magnitude":dbl[]}[])  [unwired: 1 in, 1 out]
                    }
                  }
                }
                frame True {
                  n3569 = Build Array(w5810) -> (w5809:cluster{"f0":dbl, "df":dbl, "magnitude":dbl[]}[])
                }
              }
              n3570 = for {
                tunnel: w5780 -> [w5799] mode=indexing
                tunnel: [w5798] -> w5790 mode=indexing
                workers-P: _ -> [_]
                n3571 = Unbundle By Name(w5799) -> ("magnitude"=w5798:dbl[])
              }
              n3572 = Transpose 2D Array(2D array=w5790) -> (transposed array=w5789:dbl[][])
              n3573 = for {
                tunnel: w5789 -> [w5797] mode=indexing
                tunnel: [w5796] -> w5788 mode=indexing
                workers-P: _ -> [_]
                n3574 = Add Array Elements(numeric array=w5797) -> (sum=w5796:dbl)
              }
              n3575 = Select(t=w5783, s=w5784, f=w5782) -> (s? t:f=w5781:dbl)
              n3576 = Divide(x=w5788, y=w5781) -> (x/y=w5786:dbl[])
              n3577 = Bundle By Name(cluster=w5787, "magnitude"=w5786) -> (w5785:cluster{"f0":dbl, "df":dbl, "magnitude":dbl[]})
            }
          }
        }
        n3578 = case shown="True" w5727 {
          tunnel: w5728 -> [w5759 w5765]
          tunnel: [w5759 w5760] -> w5726
          frame False {
          }
          frame True {
            n3579 = Array Subset(array=w5765, index (row)=0 ("index"), length (row)=4 ("length"), index (col)=0 ("index"), length (col)=1 ("length")) -> (w5760:T74)
          }
        }
        n3580 = feedback-in #19(w5726) -> ()
        n3581 = Split 1D Array(array=w5740, index=2) -> (first subarray=→"FFT 1":cluster{"f0":dbl, "df":dbl, "magnitude":dbl[]}[], second subarray=→"FFT 2":cluster{"f0":dbl, "df":dbl, "magnitude":dbl[]}[])
      }
    }
    n3582 = call-poly <vilib>:"Index Waveform Array.vi"("index"=16, "waveform array"=w4753) -> ("waveform"=w4776:waveform(dbl))  [unwired: 8 in, 1 out]
    n3583 = Unbundle By Name(w4776) -> ("Y"=→"PSD Y Sum":dbl[])
    n3584 = Not(x="Trap Trig. Fl.") -> (.not. x?=w4831:bool)
    n3585 = feedback-in #20("Trap Trig. Fl.") -> ()
    n3586 = feedback #20("Trap Trig. Fl.") -> (w4829:bool)
    n3587 = And(x=w4831, y=w4829) -> (x .and. y?=w4830:bool)
    n3588 = case "If have just turned off triggering" shown="True" w4830 {
      tunnel: w4769 -> [_ w5213]
      tunnel: w4825 -> [_ w5212]
      frame False {
      }
      frame True {
        w5211 = FALSE ("FPGA Trap Trig")
        n3589 = xnode "Read/Write Control"("FPGA VI Reference In"=w5213, "error in"=w5212, "FPGA Trap Trig"=w5211) -> ("FPGA VI Reference Out"=w5210:T41, "error out"=w5209:errorcluster)
        n3590 = xnode "Read/Write Control"("FPGA VI Reference In"=w5210, "error in"=w5209, "TTrig?"=w5211) -> ()  [unwired: 2 out]
        n3591 = local write "Initializing"(FALSE ("Initializing")) -> ()
        n3592 = local write "Triggered"(FALSE ("Triggered")) -> ()
        n3593 = local write "Waiting"(FALSE ("Waiting")) -> ()
      }
    }
    n3594 = Not(x=w4829) -> (.not. x?=w4842:bool)
    n3595 = And(x="Trap Trig. Fl.", y=w4842) -> (x .and. y?=w4839:bool)
    n3596 = local read "Tether"() -> (w4678:bool)
    n3597 = Or(x=w4839, y="Reinitialize") -> (x .or. y?=w4828:bool)
    n3598 = feedback #21(w4835) -> (w4840:string)
    n3599 = Select(t=w4835, s=w4839, f=w4840) -> (s? t:f=w4834:string)
    n3600 = Select(t=w4835, s="Reinitialize", f=w4834) -> (s? t:f=w4833:string)
    n3601 = feedback #22(0) -> (w4837:i32)
    n3602 = case "For determining if there is a tether still" shown="True" w4678 {
      tunnel: w4680 -> [_ w5322]
      frame False {
      }
      frame True {
        n3603 = Greater?(x="Lost Tether Alarm Threshold (pN)", y=w5322) -> (0:w5320:bool)
        n3604 = case shown="True" w5320 {
          frame False {
          }
          frame True {
            w5323 = FALSE ("Value (Signaling)")
            n3605 = flat-sequence {
              frame #0 {
                # "stop only if saving"
                n3606 = local read "Saving..."() -> (w5335:bool)
                n3607 = And(x=w5335, y="TA Cancel Save?") -> (x .and. y?=w5334:bool)
                n3608 = local write "Stop Saving"(w5334) -> ()
              }
              frame #1 {
                n3609 = case shown="True" "TA Green Off?" {
                  frame False {
                  }
                  frame True {
                    w5338 = FALSE ("Fl. Triggered...")
                    n3610 = local write "Fl. Triggered..."(w5338) -> ()
                    n3611 = property on="Vortran Laser ON" class="Bool (strict)"("Val(Sgnl)"=w5338) -> ()  [unwired: 2 in, 2 out]
                  }
                }
              }
            }
            n3612 = local read "Time tether formed"() -> (w5329:timestamp)
            n3613 = Get Date/Time In Seconds() -> (seconds since 1Jan1904=w5330:timestamp)
            n3614 = Subtract(x=w5330, y=w5329) -> (x-y=w5328:dbl)
            n3615 = Number To Decimal String(number=w5328) -> (decimal integer string=w5325:string)  [unwired: 1 out]
            n3616 = local read "Messages"() -> (w5332:string)
            n3617 = call <vilib>:"Beep.vi"() -> ()  [unwired: 3 in, 9 out]
            n3618 = Concatenate Strings("Lost tether (" ("Message to add"), w5325, " s)." ("string")) -> (w5327:string)
            n3619 = local write "Tether"(FALSE ("Tether")) -> ()
            n3620 = call "Update messages.vi"("Message to add"=w5327, "Old message string"=w5332) -> ("New message string"=w5331:string)
            n3621 = local write "Messages"(w5331) -> ()
            n3622 = property on="Fl. Triggered..." class="Bool (strict)"("Val(Sgnl)"=w5323) -> ()  [unwired: 2 in, 2 out]
            n3623 = local write "Dip for Protein"(w5323) -> ()
            n3624 = property on="Trap Pos. FB ON" class="Bool (strict)"("Val(Sgnl)"=w5323) -> ()  [unwired: 2 in, 2 out]
            n3625 = property on="Trap Trig. Fl." class="Bool (strict)"("Val(Sgnl)"=w5323) -> ()  [unwired: 2 in, 2 out]
          }
        }
      }
    }
    n3626 = case "For triggering actions based on the trap position (e.g., turning the excitation laser on if trap under feedback moves so far)" shown="True" "Trap Trig. Fl." {
      tunnel: w4717 -> [_ w5226]
      tunnel: w4833 -> [_ w5225]
      tunnel: ["" ("t") w5224] -> w4841
      tunnel: w4828 -> [_ w5223]
      tunnel: [0 ("t") w5222] -> w4838
      tunnel: w4837 -> [_ w5221]
      tunnel: w4769 -> [_ w5220]
      tunnel: w4825 -> [_ w5219]
      frame False {
      }
      frame True {
        n3627 = case shown="\"Wait for trigger\"" w5225 {
          tunnel: w5226 -> [w5243 _ _ w5291]
          tunnel: [w5240 w5272 "" ("t") w5294] -> w5224
          tunnel: w5223 -> [_ _ _ w5282]
          tunnel: [w5239 w5269 0 ("t") w5283] -> w5222
          tunnel: w5221 -> [_ w5271 _ w5289]
          tunnel: w5220 -> [w5228 w5266 _ w5285]
          tunnel: w5219 -> [w5227 w5265 _ w5284]
          frame "Wait for trigger" {
            n3628 = local read "Trap Trig. (FPGA)"() -> (w5231:bool)
            n3629 = Subtract(x=w5243, y="Mean T1 Position\nto compare (nm)") -> (x-y=w5236:dbl[])
            n3630 = call <vilib>:"Std Deviation and Variance.vi"("X"=w5236) -> ("mean"=→"mean":dbl, "standard deviation"=→"standard\ndeviation":dbl)  [unwired: 1 in, 1 out]
            n3631 = Array Max & Min(array=w5236) -> (max value=→"max value":dbl, min value=→"min value":dbl)  [unwired: 2 out]
            n3632 = Greater?(x=w5236, y="Threshold (nm)") -> (0:w5246:bool[])
            n3633 = case shown="True" w5231 {
              tunnel: w5228 -> [_ w5252]
              tunnel: w5227 -> [_ w5251]
              tunnel: [FALSE ("TTrig?") w5250] -> w5234
              frame False {
              }
              frame True {
                n3634 = xnode "Read/Write Control"("FPGA VI Reference In"=w5252, "error in"=w5251) -> ("TTrig?"=w5250:bool)  [unwired: 2 out]
              }
            }
            n3635 = Or Array Elements(Boolean array=w5246) -> (logical OR=w5233:bool)
            n3636 = Select(t=w5234, s=w5231, f=w5233) -> (s? t:f=w5232:bool)
            n3637 = Not(x=w5231) -> (.not. x?=w5230:bool)
            n3638 = And(x=w5232, y=w5230) -> (x .and. y?=w5229:bool)
            n3639 = Select(t="Triggered", s=w5232, f="Wait for trigger") -> (s? t:f=w5240:string)
            n3640 = case shown="True" w5232 {
              tunnel: [0 0] -> w5239
              tunnel: w5228 -> [_ w5257]
              tunnel: w5227 -> [_ w5256]
              frame False {
                "Waiting" <- TRUE ("Waiting")
              }
              frame True {
                n3641 = xnode "Read/Write Control"("FPGA VI Reference In"=w5257, "error in"=w5256, "TTrig?"=FALSE) -> ()  [unwired: 2 out]
                n3642 = local read "Messages"() -> (w5260:string)
                n3643 = call <vilib>:"Beep.vi"() -> ()  [unwired: 12 in]
                n3644 = call "Update messages.vi"("Message to add"="Unwinding trigger.", "Old message string"=w5260) -> ("New message string"=w5261:string)
                n3645 = local write "Messages"(w5261) -> ()
                n3646 = local write "Waiting"(FALSE ("Waiting")) -> ()
                "Triggered" <- TRUE ("Triggered")
              }
            }
            n3647 = case "Only need to turn on laser if host triggered" shown="True" w5229 {
              frame False {
              }
              frame True {
                n3648 = property on="Vortran Laser ON" class="Bool (strict)"("Val(Sgnl)"=TRUE ("Value (Signaling)")) -> ()  [unwired: 2 in, 2 out]